vi "MH.vi"() -> ()   [LabVIEW 2018] (continued)
 1.2177015412969927, 1.2175627768114623, 1.217393891699421, 1.2171947456612926, 1.2169651861682378, 1.2167050483082855, 1.216414154620753, 1.216092314918734, 1.2157393260993294, 1.2153549719413215, 1.2149390228899128, 1.214491235828264, 1.214011353835404, 1.2134991059300522, 1.2129542068000878, 1.2123763565169865, 1.211765240234963, 1.2111205278742614, 1.2104418737878937, 1.2097289164115157, 1.2089812778957194, 1.20819856372005, 1.2073803622882293, 1.2065262445038292, 1.2056357633255912, 1.2047084533017798, 1.2037438300825987, 1.2027413899099206, 1.2017006090834057, 1.200620943401988, 1.1995018275799572, 1.1983426746362595, 1.1971428752562423, 1.1959017971245343, 1.1946187842278135, 1.1932931561263076, 1.1919242071926655, 1.190511205816663, 1.1890533935745768, 1.187549984361233, 1.1860001634836392, 1.1844030867141369, 1.182757879301243, 1.1810636349367762, 1.1793194146767236, 1.1775242458142448, 1.17567712070249, 1.173776995524888, 1.1718227890107575, 1.169813381093744, 1.1677476115102279, 1.1656242783354667, 1.1634421364542267, 1.1611998959632603, 1.158896220502519, 1.1565297255115998, 1.1540989764085836, 1.151602486687458, 1.1490387159305162, 1.1464060677322425, 1.1437028875303479, 1.140927460340529, 1.13807800839016, 1.1351526886470071, 1.132149590238435, 1.129066731756324, 1.1259020584434487, 1.1226534392560812, 1.1193186637980543, 1.1158954391215752, 1.1123813863893963, 1.1087740373933732, 1.1050708309247332, 1.10126910899025, 1.0973661128703087, 1.0933589790133884, 1.0892447347624816, 1.0850202939093971, 1.0806824520726475, 1.0762278818954298, 1.0716531280609227, 1.0669546021223701, 1.062128577146724, 1.0571711821712133, 1.052078396474199, 1.0468460436618583, 1.041469785575491, 1.0359451160250122, 1.030267354357543, 1.0244316388720403, 1.0184329200946776, 1.0122659539334082, 1.0059252947339785, 0.9994052882657183, 0.9927000646697827, 0.9858035314104641, 0.9787093662768435, 0.9714110104909491, 0.9639016619883388, 0.9561742689478769, 0.9482215236600472, 0.9400358568374205, 0.9316094324858953, 0.9229341434736617, 0.9140016079541144, 0.9048031668207209, 0.8953298823956836, 0.8855725385808886, 0.8755216427280905, 0.8651674295172285, 0.8544998671643386, 0.8435086663173931, 0.8321832920359279, 0.8205129792902363, 0.8084867524560679, 0.7960934493222613, 0.7833217501687113, 0.7701602125102136, 0.756597312136108, 0.7426214911040613, 0.7282212133654118, 0.713385028708845, 0.6981016457003372, 0.6823600142717727, 0.6661494185579584, 0.6494595805017199, 0.6322807746303265, 0.614603954248466, 0.5964208890895191, 0.5777243142102709, 0.5585080896018602, 0.5387673696185277, 0.5184987808948797, 0.49770060693601686, 0.4763729770286037, 0.4545180565470823, 0.43214023513517774, 0.40924630865297024, 0.3858456502222335, 0.3619503652159427, 0.33757542465794965, 0.3127387712781067, 0.28746139243823904, 0.2617673543583629, 0.23568379255354027, 0.2092408541683436, 0.18247158896595436, 0.15541178708257433, 0.12809976325181788, 0.10057608897928992, 0.07288327602187064, 0.04506541639777282, 0.017167785914257497, -0.010763580260127775, -0.03868233023802198, -0.066542245718119, -0.09429768906113654, -0.1219040363858661, -0.14931808656186743, -0.17649843703040283, -0.2034058188067417, -0.23000338469806156, -0.2562569466125352, -0.2821351597205959, -0.3076096530569214, -0.33265510782688623, -0.3572492861418561, -0.38137301409322233, -0.4050101239745596, -0.42814736106072326, -0.4507742606709451, -0.47288300131022915, -0.49446823953357677, -0.5155269318581279, -0.5360581485996797, -0.5560628839774777, -0.5755438662488729, -0.5945053710419418, -0.6129530404680206, -0.6308937100436169, -0.6483352449424562, -0.6652863866458752, -0.6817566106622722, -0.697755995651437, -0.7132951040101064, -0.7283848737506045, -0.7430365213285615, -0.7572614549431615, -0.7710711977384661, -0.7844773202723593, -0.7974913815823875, -0.8101248781634963, -0.8223892001751673, -0.8342955942096405, -0.8458551319800632, -0.8570786843174417, -0.8679768999037287, -0.8785601882066253, -0.8888387061237083, -0.8988223478833939, -0.9085207377909621, -0.9179432254461959, -0.9270988830964301, -0.9359965048227762, -0.9446446072905432, -0.9530514318231013, -0.9612249475876249, -0.9691728557048517, -0.9769025941178192, -0.9844213430754933, -0.9917360311051868, -0.9988533413639552, -1.005779718274774, -1.012521374364737, -1.0190842972360712, -1.0254742566093968, -1.0316968113885907, -1.0377573167041594, -1.0436609308991625, -1.0494126224278009, -1.0550171766419698, -1.0604792024458223, -1.0658031388022746, -1.0709932610789714, -1.0760536872240356, -1.0809883837647403, -1.0858011716240157, -1.0904957317520383, -1.0950756105713644, -1.0995442252356191, -1.1039048687025979, -1.1081607146239931, -1.1123148220542505, -1.1163701399819441, -1.1203295116875394, -1.1241956789316945, -1.127971285978703, -1.1316588834598023, -1.135260932081046, -1.1387798061811965, -1.1422177971441378, -1.145577116671353, -1.1488598999193032, -1.1520682085066154, -1.155204033396262, -1.1582692976574447, -1.1612658591119043, -1.1641955128693555, -1.1670599937565076, -1.169860978644098, -1.172600088676191, -1.1752788914056969, -1.1778989028403013, -1.1804615894024728, -1.182968369807292, -1.1854206168615853, -1.1878196591878794, -1.1901667828763216, -1.192463233067828, -1.1947102154713283, -1.1969088978181184, -1.199060411256041, -1.2011658516860835, -1.2032262810440262, -1.2052427285294118, -1.2072161917843618, -1.209147638024209, -1.2110380051222707, -1.2128882026506116, -1.2146991128788505, -1.2164715917327598, -1.2182064697145136, -1.2199045527861077, -1.2215666232177318, -1.223193440402497, -1.2247857416390273, -1.2263442428832712, -1.2278696394709379, -1.2293626068116985, -1.230823801056524, -1.2322538597391688, -1.2336534023929442, -1.2350230311439316, -1.2363633312814712, -1.2376748718070056, -1.2389582059621622, -1.2402138717369169, -1.2414423923587334, -1.242644276763399, -1.2438200200483538, -1.24497010390929, -1.246094997060579, -1.2471951556403824, -1.248271023600837, -1.2493230330841512, -1.2503516047850498, -1.2513571483001558, -1.2523400624648429, -1.2533007356780328, -1.2542395462154847, -1.255156862531966, -1.2560530435527562, -1.2569284389549726, -1.2577833894390194, -1.2586182269906248, -1.2594332751337995, -1.2602288491750568, -1.261005256439289, -1.2617627964975509, -1.2625017613871101, -1.2632224358240298, -1.263925097408606, -1.264610016823888, -1.2652774580275623, -1.2659276784374656, -1.2665609291109212, -1.2671774549181787, -1.267777494710156, -1.2683612814806733, -1.2689290425234003, -1.2694809995837353, -1.2700173690057532, -1.2705383618744266, -1.2710441841532907, -1.271535036817718, -1.2720111159839533, -1.2724726130340556, -1.272919714736903, -1.2733526033654088, -1.2737714568100453, -1.274176448688852, -1.2745677484540103, -1.2749455214951395, -1.2753099292393857, -1.2756611292484652, -1.2759992753127154, -1.2763245175423066, -1.2766370024556426, -1.2769368730651445, -1.2772242689603854, -1.2774993263887826, -1.2777621783338409, -1.278012954591069, -1.278251781841643, -1.2784787837238858, -1.278694080902634, -1.2788977911365547, -1.279090029343509, -1.279270907663969, -1.2794405355226197, -1.2795990196881446, -1.2797464643312892, -1.2798829710812396, -1.280008639080387, -1.280123565037497, -1.280227843279383, -1.2803215658010634, -1.2804048223145295, -1.280477700296094, -1.2805402850324126, -1.2805926596651902, -1.2806349052346362, -1.2806671007216797, -1.2806893230890146, -1.2807016473209731, -1.280704146462292, -1.2806968916558, -1.2806799521790304, -1.2806533954798431, -1.280617287211024, -1.2805716912639453, -1.280516669801277, -1.2804522832888041, -1.2803785905263438, -1.2802956486778296, -1.2802035133005338, -1.28010223837352, -1.2799918763252756, -1.2798724780605988, -1.279744092986741, -1.2796067690388275, -1.2794605527045684, -1.279305489048309, -1.2791416217343863, -1.2789689930498724, -1.2787876439266608, -1.278597613962964, -1.2783989414441992, -1.2781916633633132, -1.277975815440526, -1.2777514321425336, -1.2775185467011827, -1.2772771911316114, -1.277027396249895, -1.2767691916901902, -1.2765026059214033, -1.2762276662633836, -1.2759443989026664, -1.2756528289077649, -1.275352980244028, -1.275044875788078, -1.2747285373418313, -1.2744039856461156, -1.2740712403938987, -1.273730320243124, -1.2733812428291846, -1.2730240247770153, -1.2726586817128438, -1.2722852282755772, -1.2719036781278656, -1.2715140439668149, -1.271116337534389, -1.270710569627485, -1.270296750107706, -1.2698748879108182, -1.2694449910559273, -1.269007066654354, -1.2685611209182246, -1.2681071591687978, -1.267645185844499, -1.26717520450871, -1.2666972178572817, -1.2662112277258097, -1.2657172350966377, -1.265215240105644, -1.2647052420487652, -1.2641872393883042, -1.2636612297589949, -1.2631272099738533, -1.262585176029799, -1.262035123113071, -1.2614770456044229, -1.2609109370841178, -1.2603367903367095, -1.2597545973556428, -1.259164349347635, -1.2585660367368858, -1.2579596491690832, -1.2573451755152367, -1.2567226038753156, -1.2560919215817279, -1.2554531152026018, -1.2548061705449118, -1.2541510726574292, -1.253487805833508, -1.2528163536137098, -1.2521366987882565, -1.2514488233993497, -1.2507527087433046, -1.250048335372562, -1.2493356830975233, -1.2486147309882596, -1.2478854573760618, -1.2471478398548568, -1.246401855282477, -1.2456474797817987, -1.244884688741737, -1.2441134568181147, -1.2433337579343902, -1.2425455652822728, -1.2417488513221855, -1.2409435877836272, -1.2401297456653948, -1.239307295235693, -1.238476206032117, -1.2376364468615264, -1.236787985799793, -1.235930790191438, -1.235064826649166, -1.2341900610532692, -1.2333064585509415, -1.2324139835554728, -1.2315125997453407, -1.2306022700632027, -1.22968295671478, -1.2287546211676412, -1.2278172241498915, -1.2268707256487568, -1.2259150849090803, -1.224950260431717, -1.2239762099718374, -1.2229928905371452, -1.2220002583859966, -1.2209982690254362, -1.2199868772091478, -1.2189660369353148, -1.2179357014444019, -1.2168958232168547, -1.215846353970713, -1.2147872446591514, -1.213718445467943, -1.2126399058128463, -1.2115515743369103, -1.2104533989077249, -1.2093453266145828, -1.2082273037655835, -1.207099275884668, -1.2059611877085838, -1.2048129831837935, -1.2036546054633184, -1.2024859969035147, -1.2013070990608123, -1.200117852688371, -1.1989181977327046, -1.197708073330238, -1.1964874178038265, -1.1952561686592202, -1.1940142625814778, -1.1927616354313497, -1.1914982222416113, -1.1902239572133557, -1.1889387737122594, -1.1876426042647972, -1.1863353805544512, -1.1850170334178567, -1.1836874928409564, -1.182346687955106, -1.1809945470331706, -1.1796309974855963, -1.1782559658564766, -1.1768693778195976, -1.1754711581744743, -1.17406123084239, -1.172639518862421, -1.1712059443874778, -1.1697604286803325, -1.1683028921096728, -1.1668332541461484, -1.165351433358459, -1.163857347409433, -1.1623509130521548, -1.1608320461261021, -1.1593006615533306, -1.1577566733346853, -1.1561999945460588, -1.1546305373346903, -1.153048212915527, -1.1514529315676323, -1.1498446026306577, -1.1482231345013842, -1.1465884346303372, -1.1449404095184774, -1.1432789647139758, -1.1416040048090828, -1.1399154334370947, -1.1382131532694137, -1.1364970660127376, -1.1347670724063428, -1.1330230722195127, -1.1312649642490857, -1.1294926463171435, -1.1277060152688512, -1.1259049669704502, -1.1240893963074112, -1.1222591971827605, -1.1204142625155937, -1.118554484239768, -1.1166797533028008, -1.114789959664974, -1.11288499229866, -1.1109647391878672, -1.1090290873280393, -1.1070779227260887, -1.1051111304006993, -1.1031285943828988, -1.10113019771692, -1.0991158224613446, -1.097085349690569, -1.0950386594965857, -1.0929756309910947, -1.0908961423079597, -1.0888000706060428, -1.0866872920723838, -1.0845576819258087, -1.0824111144208897, -1.0802474628523797, -1.0780665995600416, -1.075868395933946, -1.0736527224202304, -1.0714194485273458, -1.0691684428328063, -1.066899572990445, -1.0646127057382266, -1.0623077069065903, -1.0599844414273953, -1.0576427733434381, -1.0552825658185843, -1.0529036811485564, -1.0505059807723431, -1.0480893252843075, -1.045653574446987, -1.0431985872046041, -1.0407242216973305, -1.0382303352763054, -1.0357167845194528, -1.0331834252480923, -1.0306301125444122, -1.028056700769775, -1.0254630435839351, -1.0228489939651428, -1.0202144042312107, -1.0175591260615238, -1.0148830105200592, -1.0121859080794056, -1.0094676686458401, -1.0067281415854912, -1.0039671757515733, -1.0011846195127831, -0.9983803207828486, -0.9955541270512621, -0.9927058854152399, -0.9898354426129405, -0.9869426450579505, -0.9840273388750918, -0.9810893699375822, -0.9781285839055489, -0.9751448262659631, -0.9721379423740234, -0.9691077774959831, -0.9660541768535129, -0.9629769856695575, -0.9598760492158033, -0.956751212861706, -0.9536023221251739, -0.9504292227249033, -0.9472317606344008, -0.9440097821377474, -0.9407631338871011, -0.9374916629619968, -0.9341952169304646, -0.9308736439119777, -0.9275267926423061, -0.9241545125402463, -0.9207566537763047, -0.9173330673433207, -0.9138836051291086, -0.9104081199910655, -0.9069064658328728, -0.9033784976831947, -0.8998240717765209, -0.8962430456360665, -0.8926352781588002, -0.8890006297026586, -0.8853389621758396, -0.8816501391283417, -0.8779340258456287, -0.8741904894445335, -0.870419398971334, -0.8666206255020502, -0.8627940422449536, -0.8589395246452829, -0.8550569504921887, -0.8511462000278703, -0.8472071560589071, -0.8432397040698157, -0.8392437323387362, -0.8352191320553193, -0.8311657974407253, -0.8270836258697578, -0.8229725179950594, -0.8188323778733954, -0.8146631130939137, -0.8104646349084322, -0.8062368583636034, -0.8019797024349924, -0.7976930901629831, -0.7933769487904367, -0.7890312099020518, -0.7846558095653562, -0.78025068847327, -0.7758157920881004, -0.7713510707869703, -0.7668564800085034, -0.7623319804007153, -0.7577775379699825, -0.7531931242310075, -0.7485787163576143, -0.7439342973342988, -0.7392598561083555, -0.7345553877425073, -0.7298208935678053, -0.7250563813367559, -0.7202618653763987, -0.7154373667412799, -0.7105829133660783, -0.7056985402177304, -0.70078428944689, -0.6958402105384889, -0.6908663604612254, -0.6858628038158068, -0.6808296129816426, -0.6757668682619226, -0.6706746580266866, -0.6655530788537816, -0.6604022356674474, -0.6552222418742362, -0.6500132194961148, -0.6447752993003919, -0.6395086209263622, -0.6342133330082297, -0.6288895932942323, -0.6235375687615593, -0.6181574357269265, -0.6127493799523775, -0.6073135967462472, -0.6018502910588119, -0.5963596775725288, -0.5908419807864443, -0.5852974350946539, -0.5797262848583801, -0.574128784471564, -0.5685051984195624, -0.5628558013308195, -0.5571808780211295, -0.5514807235303619, -0.5457556431513001, -0.5400059524504468, -0.5342319772804425, -0.528434053784033, -0.5226125283892138, -0.5167677577954828, -0.5109001089508638, -0.505009959019655, -0.4990976953406679, -0.49316371537574794, -0.48720842664855235, -0.48123224667332604, -0.4752356028736789, -0.4692189324911475, -0.46318268248357125, -0.457127309413122, -0.45105327932403533, -0.4449610676098665, -0.43885115887047843, -0.432724046758543, -0.4265802338157381, -0.42042023129863165, -0.4142445589943362, -0.40805374502599634, -0.40184832564828527, -0.395628845032946, -0.3893958550446411, -0.383149915007224, -0.3768915914605855, -0.3706214579084225, -0.364340094557028, -0.3580480880454829, -0.35174603116739545, -0.345434522584651, -0.3391141665333365, -0.3327855725222741, -0.326449355024483, -0.3201061331619721, -0.3137565303841797, -0.30740117414057805, -0.3010406955477559, -0.29467572905149236, -0.28830691208421905, -0.28193488471834594, -0.27556028931592425, -0.26918377017516226, -0.2628059731741481, -0.25642754541249785, -0.2500491348511651, -0.24367138995117796, -0.23729495931156602, -0.23092049130721934, -0.22454863372697326, -0.21818003341261857, -0.21181533589920318, -0.20545518505716698, -0.19910022273690556, -0.19275108841608654, -0.18640841885034204, -0.18007284772772922, -0.17374500532750017, -0.16742551818355317, -0.16111500875308196, -0.15481409509080446, -0.14852339052923091, -0.14224350336528807, -0.1359750365538439, -0.12971858740828734, -0.12347474730873174, -0.11724410141797262, -0.11102722840569672, -0.10482470018110408, -0.09863708163426094, -0.0924649303864426, -0.08630879654973529, -0.08016922249600472, -0.07404674263553336, -0.06794188320541796, -0.06185516206794708, -0.055787088518998565, -0.049738163106634876, -0.04370887745995003, -0.03769971412824787, -0.03171114643054984, -0.025743638315537033, -0.019797644231837032, -0.013873609008722754, -0.00797196774711847, -0.002093145720915979, 0.0037624417114971815, 0.00959438918560385, 0.01540230139906713, 0.021185793170152824, 0.02694448948638101, 0.03267802554357185, 0.03838604677537955, 0.044068208873632816, 0.04972417779948121, 0.05535362978572166, 0.06095625133038307, 0.06653173918187127, 0.07207980031585322, 0.07760015190413408, 0.08309252127575234, 0.08855664587057181, 0.09399227318558757]] ("return value 3") -> [_ w1059]
                  tunnel: "3.6" ("Python version") -> [w1017 w1058]
                  tunnel: w1003 -> [_ w1056]
                  tunnel: w1002 -> [_ w1055]
                  tunnel: w1001 -> [_ w1054]
                  tunnel: w1000 -> [_ w1053]
                  tunnel: w999 -> [_ w1052]
                  tunnel: w998 -> [_ w1051]
                  tunnel: w997 -> [_ w1050]
                  tunnel: w996 -> [_ w1049]
                  tunnel: w995 -> [_ w1048]
                  tunnel: w994 -> [_ w1047]
                  tunnel: w993 -> [_ w1046]
                  tunnel: w992 -> [_ w1045]
                  tunnel: w991 -> [_ w1044]
                  tunnel: w990 -> [_ w1043]
                  tunnel: w989 -> [_ w1042]
                  tunnel: w988 -> [_ w1040]
                  frame "Read data from a g-factor file", Default {
                    n276 = Open Python Session(python version=w1017) -> (session out=w1031:refnum<k35>, error out=w1029:errorcluster)  [unwired: 2 in]
                    n277 = node(w1031, w1016, "ReadDataFunctionName 2", w1029, cluster{dbl[], dbl[]}[] [], "Date 2", "Time 2", "Filepath Name 2", "Coil") -> (w1030:refnum<k35>, w1028:errorcluster, w1020:cluster{dbl[], dbl[]}[])  [unwired: 4 in, 2 out]
                    n278 = Index Array(array=w1020, index #1=0 ("index (row)")) -> (element #1=w1019:cluster{dbl[], dbl[]}, element #2=w1018:cluster{dbl[], dbl[]})  [unwired: 1 in]
                    n279 = Close Python Session(session in=w1030, error in=w1028) -> (11:→"readG-FactorFilesError  2":errorcluster)
                  }
                  frame "Calculate G-factor" {
                    n280 = Concatenate Strings(w1040, "\\\\Mcoil") -> (w1034:string)
                    n281 = case shown="\"Simulation\", Default" w1062 {
                      tunnel: w1072 -> [w1089 w1116]
                      tunnel: [w1090 w1115] -> w1063
                      tunnel: w1047 -> [w1086 _]
                      tunnel: w1046 -> [w1085 _]
                      tunnel: w1045 -> [w1084 _]
                      tunnel: w1044 -> [w1083 _]
                      tunnel: w1043 -> [w1082 _]
                      tunnel: w1061 -> [w1081 _]
                      tunnel: w1049 -> [w1080 w1104]
                      tunnel: w1048 -> [w1079 w1103]
                      tunnel: w1050 -> [w1078 w1102]
                      tunnel: w1056 -> [_ w1110]
                      tunnel: w1055 -> [_ w1109]
                      tunnel: w1054 -> [_ w1108]
                      tunnel: w1053 -> [_ w1107]
                      tunnel: w1052 -> [_ w1106]
                      tunnel: w1051 -> [_ w1105]
                      tunnel: w1060 -> [w1087 w1114]
                      tunnel: w1059 -> [w1092 w1113]
                      tunnel: w1058 -> [w1088 w1112]
                      tunnel: [w1091 w1111] -> w1057
                      tunnel: w1034 -> [w1077 w1101]
                      tunnel: w1042 -> [w1076 w1100]
                      tunnel: [w1075 w1099] -> w1033
                      tunnel: "function name gfactor 2" -> [w1073 w1097]
                      frame "Simulation", Default {
                        n282 = Open Python Session(python version=w1088) -> (session out=w1096:refnum<k35>, error out=w1094:errorcluster)  [unwired: 2 in]
                        n283 = node(w1096, w1087, w1073, w1094, w1092, w1086, w1085, w1084, w1083, w1082, w1081, w1080, w1079, w1078, w1089, w1077, w1076) -> (w1095:refnum<k35>, w1093:errorcluster, w1090:dbl[][])  [unwired: 12 in, 2 out]
                        n284 = Close Python Session(session in=w1095, error in=w1093) -> (11:w1091:errorcluster)
                        n285 = Concatenate Strings(w1076, "Used coil parameters from manual fit to calculate gfactor" ("filename")) -> (w1075:string)
                      }
                      frame "Fit" {
                        n286 = Open Python Session(python version=w1112) -> (session out=w1120:refnum<k35>, error out=w1118:errorcluster)  [unwired: 2 in]
                        n287 = node(w1120, w1114, w1097, w1118, w1113, w1110, w1109, w1108, w1107, w1106, w1105, w1104, w1103, w1102, w1116, w1101, w1100) -> (w1119:refnum<k35>, w1117:errorcluster, w1115:dbl[][])  [unwired: 12 in, 2 out]
                        n288 = Close Python Session(session in=w1119, error in=w1117) -> (11:w1111:errorcluster)
                        n289 = Concatenate Strings(w1100, "Used coil parameters from automatic fit to calculate gfactor" ("filename")) -> (w1099:string)
                      }
                    }
                    "return value gM" <- w1063
                    "gfactor M: error out" <- w1057
                    n290 = String To Path(string=w1034) -> (path=w1035:path)
                    n291 = Index Array(array=w1063, index (row) #1=0, index (row) #2=1 ("index (page)"), index (row) #3=2 ("index (page)")) -> (element #1=w1066:dbl[], element #2=w1068:dbl[], element #3=w1067:dbl[])  [unwired: 3 in]
                    n292 = Concatenate Strings(w1033, ".txt") -> (w1038:string)
                    n293 = Bundle("return value 3"=w1066, "return value 3"=w1068) -> (w1065:T6)  [unwired: 1 in]
                    n294 = Bundle("return value 3"=w1066, "return value 3"=w1067) -> (w1064:T6)  [unwired: 1 in]
                    n295 = Build Path(base path=w1035, name or relative path=w1038) -> (appended path=w1037:path)
                    n296 = Write to Text File(file (use dialog)=w1037, text=" " ("file content")) -> ()  [unwired: 2 in, 3 out]
                  }
                }
                "gfactor M (magnitude)" <- w1012
                "gfactor M (phase)" <- w1011
              }
            }
          }
          frame "Voltage and Temp Data Display Panel" {
            n297 = case shown="True" "?" {
              tunnel: w1122 -> [_ w1135]
              tunnel: w1121 -> [_ w1134]
              frame False {
              }
              frame True {
                n298 = case shown="\"Measure:\", Default" "Voltage data source:" {
                  tunnel: w1135 -> [w1160 _]
                  tunnel: w1134 -> [w1159 _]
                  tunnel: "ModulePath" -> [w1156 w1174]
                  tunnel: [w1148 w1185] -> w1132
                  tunnel: [w1147 w1184] -> w1131
                  tunnel: [w1146 w1173] -> w1130
                  frame "Measure:", Default {
                    n299 = Open Python Session(python version="3.6" ("Python version")) -> (session out=w1158:refnum<k35>, error out=w1154:errorcluster)  [unwired: 2 in]
                    n300 = Boolean To (0,1)(Boolean="Run Checkscale?") -> (0, 1=w1139:i16)
                    n301 = Boolean To (0,1)(Boolean="Run with Simulator") -> (0, 1=w1141:i16)
                    n302 = node(w1158, w1156, "mainForAmbrell", w1154, cluster{"Array 2":dbl[], "Array 3":dbl[]}[][] [[{"Array 2"=array[100000 elements], "Array 3"=array[100000 elements]}, {"Array 2"=array[100000 elements], "Array 3"=array[100000 elements]}, {"Array 2"=array[100000 elements], "Array 3"=array[100000 elements]}]] ("Array 2"), "shortRecordLength", "longRecordLength 2", "scopeNumCollects", "numChan", "Operating Frequency of EASYHEAT", w1139, w1160, w1159, "Run", w1141) -> (w1152:refnum<k35>, w1153:errorcluster, w1149:cluster{"Array 2":dbl[], "Array 3":dbl[]}[][], w1138:i64)  [unwired: 9 in, 2 out]
                    n303 = Increment(x=w1138) -> (x+1=w1137:i64)
                    n304 = local write "Run"(w1137) -> ()
                    n305 = Close Python Session(session in=w1152, error in=w1153) -> (11:→"mainForAmbrellError":errorcluster)
                    n306 = Index Array(array=w1149, index (row) #1=0 ("index (page)"), index (row) #2=1 ("index (page)"), index (row) #3=2 ("index (page)")) -> (element #1=w1148:cluster{"Array 2":dbl[], "Array 3":dbl[]}[], element #2=w1147:cluster{"Array 2":dbl[], "Array 3":dbl[]}[], element #3=w1146:cluster{"Array 2":dbl[], "Array 3":dbl[]}[])  [unwired: 3 in]
                  }
                  frame "From data file:" {
                    n307 = Open Python Session(python version="3.6" ("Python version")) -> (session out=w1182:refnum<k35>, error out=w1181:errorcluster)  [unwired: 2 in]
                    n308 = while {
                      tunnel: [w1216] -> w1190
                      tunnel: [w1215] -> w1189
                      tunnel: w1174 -> [w1214]
                      tunnel: [w1212] -> w1186
                      tunnel: "readDataFileVoltageName" -> [w1211]
                      tunnel: w1182 -> [w1210]
                      tunnel: w1181 -> [w1209]
                      tunnel: "dataFilePath" -> [w1207]
                      tunnel: "Time" -> [w1206]
                      tunnel: "Date" -> [w1205]
                      tunnel: "Run" -> [w1203]
                      stop <- TRUE stop-if-true
                      n309 = node(w1210, w1214, w1211, w1209, cluster{"Array 2":dbl[], "Array 3":dbl[]}[][] [[{"Array 2"=array[100000 elements], "Array 3"=array[100000 elements]}, {"Array 2"=array[100000 elements], "Array 3"=array[100000 elements]}, {"Array 2"=array[100000 elements], "Array 3"=array[100000 elements]}]] ("Array 2"), w1207, w1205, w1206, "numChan 2", w1203) -> (w1215:refnum<k35>, w1216:errorcluster, w1212:cluster{"Array 2":dbl[], "Array 3":dbl[]}[][])  [unwired: 5 in, 2 out]
                    }
                    n310 = Open Python Session(python version="3.6" ("Python version")) -> (session out=w1179:refnum<k35>, error out=w1177:errorcluster)  [unwired: 2 in]
                    n311 = while {
                      tunnel: w1179 -> [w1202]
                      tunnel: [w1201] -> w1178
                      tunnel: w1177 -> [w1200]
                      tunnel: [w1199] -> w1176
                      tunnel: w1174 -> [w1198]
                      tunnel: [w1196] -> w1173
                      tunnel: "readDataFileTemperatureName" -> [w1195]
                      tunnel: "dataFilePath" -> [w1193]
                      tunnel: "Time" -> [w1192]
                      tunnel: "Date" -> [w1191]
                      stop <- TRUE stop-if-true
                      n312 = node(w1202, w1198, w1195, w1200, cluster{"Array 2":dbl[], "Array 3":dbl[]}[] [{"Array 2"=array[100000 elements], "Array 3"=array[100000 elements]}, {"Array 2"=array[100000 elements], "Array 3"=array[100000 elements]}, {"Array 2"=array[100000 elements], "Array 3"=array[100000 elements]}] ("Array 2"), w1193, w1191, w1192) -> (w1201:refnum<k35>, w1199:errorcluster, w1196:cluster{"Array 2":dbl[], "Array 3":dbl[]}[])  [unwired: 3 in, 2 out]
                    }
                    n313 = Index Array(array=w1186, index (row) #1=0 ("index (page)")) -> (element #1=w1185:cluster{"Array 2":dbl[], "Array 3":dbl[]}[], element #2=w1184:cluster{"Array 2":dbl[], "Array 3":dbl[]}[])  [unwired: 5 in, 1 out]
                    n314 = Close Python Session(session in=w1189, error in=w1190) -> (11:→"readDataFileVoltageError":errorcluster)
                    n315 = Close Python Session(session in=w1178, error in=w1176) -> (11:→"readDataFileTempError":errorcluster)
                  }
                }
                "Oscilloscope Channel 1 Output Graph" <- w1132
                "Oscilloscope Channel 2 Output Graph" <- w1131
                "Opsens Channel 1" <- w1130
              }
            }
          }
          frame "Analyze: MH" {
          }
          frame "Save data/report to Excel" {
          }
        }
        n316 = Wait (ms)(milliseconds to wait=u32 100) -> ()  [unwired: 1 out]
      }
    }
  }